vi "detectFly.vi"(4 "focus check":T2=refnum, 5 "im proc controls":T1={"Color Plane"=2, "downsampling"=24, "Filter"=enum."AutoM", "Number of Erosions"=2, "Focus threshold"=20.0, "Focus std threshold"=0.0, "background\nsubtraction"=FALSE, "Threshold"=0} {"Threshold" scale=0.0..255.0; "Color Plane" items=["Red", "Green", "Blue", "Hue", "Saturation", "Luminance", "Value", "Intensity"]}, 6 "processed image container":T2=refnum caption="processed", 7 "cropped image":T2=refnum caption="cropped", 8 "raw image container":T2=refnum caption="raw") -> (0 "acquired FPS":dbl=23.880597014925375, 1 "processed image":T2, 2 "processed FPS":dbl=23.880597014925375, 3 "raw out":T2)   [LabVIEW 2012]
uses:
  <vilib>/vision/Image Controls.llb/IMAQ Image.ctl
  GlobalBaslerCamera.vi
  <vilib>/vision/driver/NI_Vision_Acquisition_Software.lvlib
  <vilib>/vision/NI_Vision_Development_Module.lvlib
panel:
  out "Global Report":T3={"Mean Value"=1.2830653, "Standard Variation"=7.5779014, "Minimal Value"=0.0, "Maximal Value"=151.0, "Area (calibrated)"=1470000.0, "Area (pixels)"=1470000, "%"=100.0, "Calibration Valid"=TRUE} {"Mean Value" format="%.2f"; "%" format="%.2f"; "Area (calibrated)" format="%.2f"; "Maximal Value" format="%.2f"; "Minimal Value" format="%.2f"; "Standard Variation" format="%.2f"}
  out "Buffer Number Out":u32=414
  out "Number of Particles":i32=1
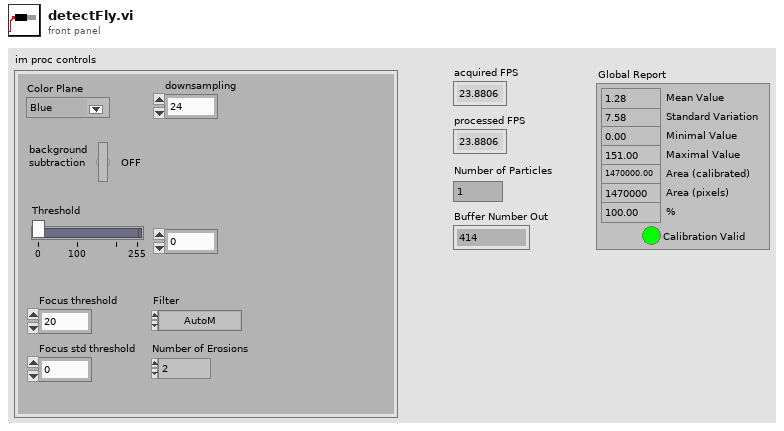
[diagram p1: front panel]
types:
  T1 = cluster{"Color Plane":i32, "downsampling":i32, "Filter":enum32{"AutoM", "Close", "Dilate", "Erode", "Gradient", "Gradient out", "Gradient in", "Hit miss", "Open", "PClose", "POpen", "Thick", "Thin"}, "Number of Erosions":i32, "Focus threshold":sgl, "Focus std threshold":sgl, "background\nsubtraction":bool, "Threshold":u8}
  T2 = typedef "IMAQ Image.ctl" = refnum<image>
  T3 = cluster{"Mean Value":sgl, "Standard Variation":sgl, "Minimal Value":sgl, "Maximal Value":sgl, "Area (calibrated)":sgl, "Area (pixels)":u32, "%":sgl, "Calibration Valid":bool}
  T4 = typedef "IMAQdx.ctl" = refnum<k21>
  T5 = enum32{"Differentiation", "Gradient", "Prewitt", "Roberts", "Sigma", "Sobel"}
  T6 = enum32{"AutoM", "Close", "Dilate", "Erode", "Gradient", "Gradient out", "Gradient in", "Hit miss", "Open", "PClose", "POpen", "Thick", "Thin"}
  T7 = typedef "Particle Parameters" = i32
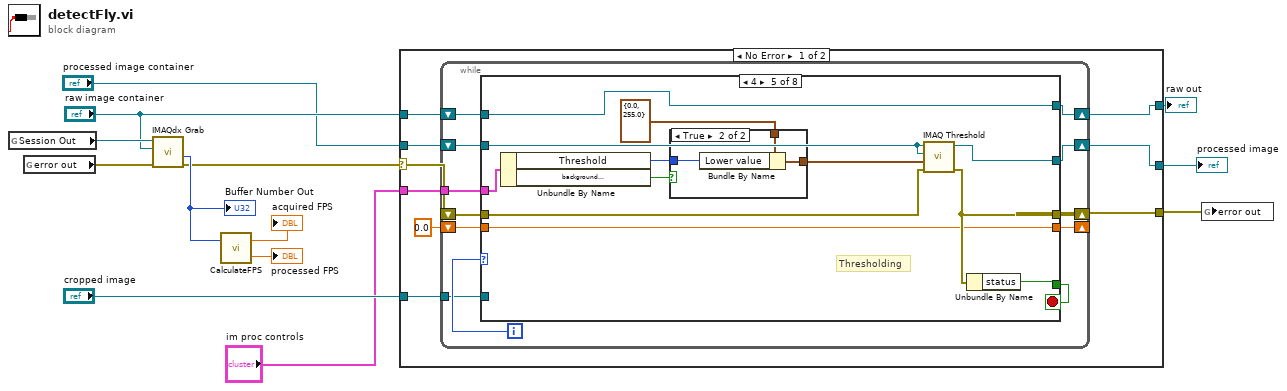
[diagram p0: block diagram]
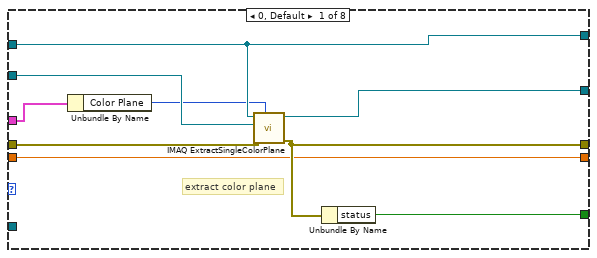
[diagram p2: hidden frame]
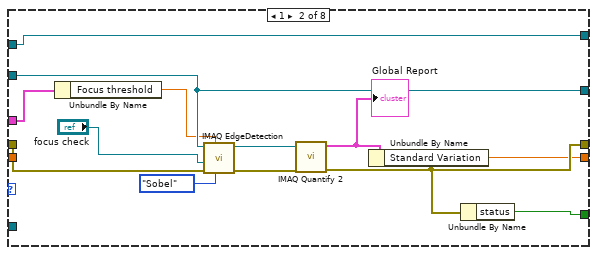
[diagram p3: hidden frame]
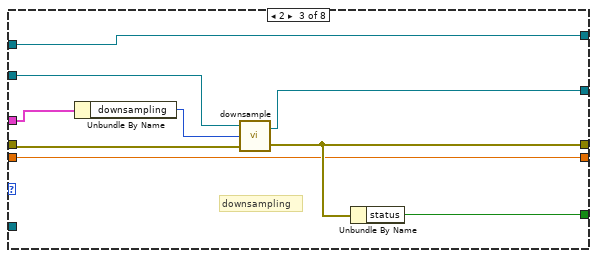
[diagram p4: hidden frame]
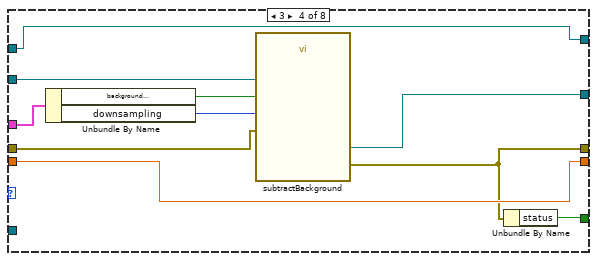
[diagram p5: hidden frame]
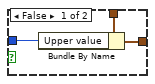
[diagram p6: hidden frame]
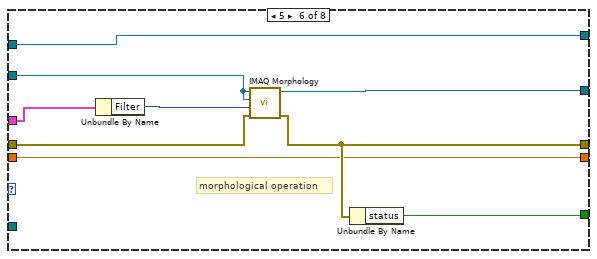
[diagram p7: hidden frame]
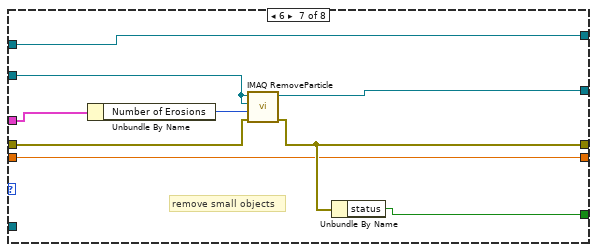
[diagram p8: hidden frame]
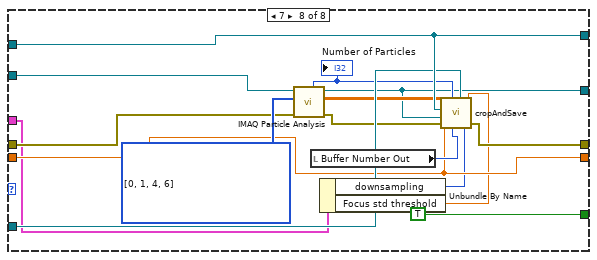
[diagram p9: hidden frame]
diagram:
  n1 = global read "GlobalBaslerCamera.vi" "Session Out"() -> (w13:T4)
  n2 = global read "GlobalBaslerCamera.vi" "error out"() -> (w12:errorcluster)
  n3 = call <vilib>:"IMAQdx Grab.vi"("error in"=w12, "Image In"="raw image container", "Session In"=w13) -> ("error out"=w9:errorcluster, "Buffer Number Out"=w11:u32)  [unwired: 1 in, 6 out]
  "Buffer Number Out" <- w11
  n4 = call "CalculateFPS.vi"("buffer number"=w11) -> ("processed FPS"=→"processed FPS":dbl, "acquired FPS"=→"acquired FPS":dbl)  [unwired: 1 in]
  n5 = case shown="No Error" w9 {
    selector: w9 -> [w22 w129]
    tunnel: "raw image container" -> [w21 w128]
    tunnel: "processed image container" -> [w20 w130]
    tunnel: [w19 w130] -> w6
    tunnel: [w18 w129] -> w4
    tunnel: [w17 w128] -> w5
    tunnel: "cropped image" -> [w16 _]
    tunnel: "im proc controls" -> [w14 _]
    frame No Error {
      n6 = while {
        shift-right: [w32] -> w18
        shift-left: w22 -> [w29]
        tunnel: w16 -> [w27]
        shift-right: [w26] -> _
        shift-left: sgl 0.0 ("Standard Variation") -> [w25]
        tunnel: w14 -> [w24]
        shift-right: [w28] -> w17
        shift-left: w21 -> [w31]
        shift-right: [w23] -> w19
        shift-left: w20 -> [w30]
        i -> [w34]
        stop <- w33 stop-if-true
        n7 = case shown="4" w34 {
          tunnel: [w40 w51 w63 w74 w85 w101 w109 TRUE ("status")] -> w33
          tunnel: [w41 w50 w62 w66 w84 w100 w108 w120] -> w32
          tunnel: w31 -> [w38 w52 w60 w73 w76 w97 w106 w123]
          tunnel: w30 -> [w43 w49 w64 w71 w87 w99 w111 w127]
          tunnel: w29 -> [w42 w47 w65 w68 w86 w102 w110 w125]
          tunnel: [w39 w49 w61 w67 w83 w98 w107 w116] -> w23
          tunnel: [w38 w52 w60 w73 w76 w97 w106 w123] -> w28
          tunnel: w27 -> [_ _ _ _ _ _ _ w122]
          tunnel: [w37 w46 w59 w72 w82 w96 w105 w115] -> w26
          tunnel: w25 -> [w37 _ w59 w72 w82 w96 w105 w115]
          tunnel: w24 -> [w36 w45 w58 w75 w78 w94 w104 w113]
          frame 0, Default {
            # "extract color plane"
            n8 = Unbundle By Name(w36) -> ("Color Plane"=w35:i32)
            n9 = call "IMAQ ExtractSingleColorPlane"("Color Plane"=w35, "error in (no error)"=w42, "Image Dst"=w43, "Image Src"=w38) -> ("error out"=w41:errorcluster, "Image Dst Out"=w39:T2)  [unwired: 6 in]
            n10 = Unbundle By Name(w41) -> ("status"=w40:bool)
          }
          frame 1 {
            n11 = Unbundle By Name(w45) -> ("Focus threshold"=w44:sgl)
            n12 = call "IMAQ EdgeDetection"("Method"=T5."Sobel", "Threshold Value"=w44, "error in (no error)"=w47, "Image Dst"="focus check", "Image Src"=w49) -> ("error out"=w55:errorcluster, "Image Dst Out"=w54:T2)  [unwired: 5 in]
            n13 = call "IMAQ Quantify 2"("error in (no error)"=w55, "Image"=w54) -> ("error out"=w50:errorcluster, "Global Report"=w53:T3)  [unwired: 7 in, 1 out]
            "Global Report" <- w53
            n14 = Unbundle By Name(w53) -> ("Standard Variation"=w46:sgl)
            n15 = Unbundle By Name(w50) -> ("status"=w51:bool)
          }
          frame 2 {
            # "downsampling"
            n16 = Unbundle By Name(w58) -> ("downsampling"=w57:i32)
            n17 = call "downsample.vi"("error in"=w65, "downsampling"=w57, "IMAQImage"=w64) -> ("error out"=w62:errorcluster, "Image Dst Out"=w61:T2)
            n18 = Unbundle By Name(w62) -> ("status"=w63:bool)
          }
          frame 3 {
            n19 = Unbundle By Name(w75) -> ("background\nsubtraction"=w70:bool, "downsampling"=w69:i32)
            n20 = call "subtractBackground.vi"("error IO"=w68, "downsampling"=w69, "saveBG"=w70, "processed image"=w71) -> ("error out"=w66:errorcluster, "processed image out"=w67:T2)  [unwired: 6 in]
            n21 = Unbundle By Name(w66) -> ("status"=w74:bool)
          }
          frame 4 {
            # "Thresholding"
            n22 = Unbundle By Name(w78) -> ("Threshold"=w81:u8, "background\nsubtraction"=w77:bool)
            n23 = case shown="True" w77 {
              tunnel: w81 -> [w90 w93]
              tunnel: [w89 w92] -> w80
              tunnel: cluster{"Lower value":sgl, "Upper value":sgl} {"Lower value"=0.0, "Upper value"=255.0} ("Range") -> [w88 w91]
              frame False {
                n24 = Bundle By Name(cluster=w88, "Upper value"=w90) -> (w89:cluster{"Lower value":sgl, "Upper value":sgl})
              }
              frame True {
                n25 = Bundle By Name(cluster=w91, "Lower value"=w93) -> (w92:cluster{"Lower value":sgl, "Upper value":sgl})
              }
            }
            n26 = call "IMAQ Threshold"("error in (no error)"=w86, "Range"=w80, "Image Dst"=w87, "Image Src"=w87) -> ("error out"=w84:errorcluster, "Image Dst Out"=w83:T2)  [unwired: 6 in]
            n27 = Unbundle By Name(w84) -> ("status"=w85:bool)
          }
          frame 5 {
            # "morphological operation"
            n28 = Unbundle By Name(w94) -> ("Filter"=w95:T6)
            n29 = call "IMAQ Morphology"("error in (no error)"=w102, "Operation"=w95, "Image Dst"=w99, "Image Src"=w99) -> ("error out"=w100:errorcluster, "Image Dst Out"=w98:T2)  [unwired: 6 in]
            n30 = Unbundle By Name(w100) -> ("status"=w101:bool)
          }
          frame 6 {
            # "remove small objects"
            n31 = Unbundle By Name(w104) -> ("Number of Erosions"=w103:i32)
            n32 = call "IMAQ RemoveParticle"("error in (no error)"=w110, "Number of Erosion"=w103, "Image Dst"=w111, "Image Src"=w111) -> ("error out"=w108:errorcluster, "Image Dst Out"=w107:T2)  [unwired: 6 in]
            n33 = Unbundle By Name(w108) -> ("status"=w109:bool)
          }
          frame 7 {
            w126 = T7[] [0, 1, 4, 6] items=["Center of Mass X", "Center of Mass Y", "First Pixel X", "First Pixel Y", "Bounding Rect Left", "Bounding Rect Top", "Bounding Rect Right", "Bounding Rect Bottom", "Max Feret Diameter Start X", "Max Feret Diameter Start Y", "Max Feret Diameter End X", "Max Feret Diameter End Y", "Max Horiz. Segment Length Left", "Max Horiz. Segment Length Right", "Max Horiz. Segment Length Row", "-", "Bounding Rect Width", "Bounding Rect Height", "Bounding Rect Diagonal", "Perimeter", "Convex Hull Perimeter", "Holes' Perimeter", "Max Feret Diameter", "Equivalent Ellipse Major Axis", "Equivalent Ellipse Minor Axis", "Equivalent Ellipse Minor Axis (Feret)", "Equivalent Rect Long Side", "Equivalent Rect Short Side", "Equivalent Rect Diagonal", "Equivalent Rect Short Side (Feret)", "Average Horiz. Segment Length", "Average Vert. Segment Length", "Hydraulic Radius", "Waddel Disk Diameter", "-", "Area", "Holes' Area", "Particle & Holes' Area", "Convex Hull Area", "Image Area", "-", "Number of Holes", "Number of Horiz. Segments", "Number of Vert. Segments", "-", "Orientation", "Max Feret Diameter Orientation", "-", "% Area/Image Area", "% Area/(Particle & Holes' Area)", "Ratio of Equivalent Ellipse Axes", "Ratio of Equivalent Rect Sides", "-", "Elongation Factor", "Compactness Factor", "Heywood Circularity Factor", "Type Factor", "-", "Sum X", "Sum Y", "Sum XX", "Sum XY", "Sum YY", "Sum XXX", "Sum XXY", "Sum XYY", "Sum YYY", "-", "Moment of Inertia XX", "Moment of Inertia XY", "Moment of Inertia YY", "Moment of Inertia XXX", "Moment of Inertia XXY", "Moment of Inertia XYY", "Moment of Inertia YYY", "Norm. Moment of Inertia XX", "Norm. Moment of Inertia XY", "Norm. Moment of Inertia YY", "Norm. Moment of Inertia XXX", "Norm. Moment of Inertia XXY", "Norm. Moment of Inertia XYY", "Norm. Moment of Inertia YYY", "Hu Moment 1", "Hu Moment 2", "Hu Moment 3", "Hu Moment 4", "Hu Moment 5", "Hu Moment 6", "Hu Moment 7"] ("Pixel Measurements")
            n34 = call "IMAQ Particle Analysis"("error in (no error)"=w125, "Pixel Measurements"=w126, "Image"=w127) -> ("error out"=w121:errorcluster, "Particle Measurements (Pixels)"=w119:dbl[][], "Image Out (duplicate)"=w116:T2, "Number of Particles"=w118:i32)  [unwired: 2 in, 3 out]
            "Number of Particles" <- w118
            n35 = local read "Buffer Number Out"() -> (w117:u32)
            n36 = Unbundle By Name(w113) -> ("downsampling"=w114:i32, "Focus std threshold"=w112:sgl)
            n37 = call "cropAndSave.vi"("error in (no error)"=w121, "downsampling"=w114, "std threshold"=w112, "cropped Image"=w122, "buffer number"=w117, "Standard Variation"=w115, "processed image"=w116, "Number of Particles"=w118, "raw image"=w123, "Particle Measurements (Pixels)"=w119) -> ("error out"=w120:errorcluster)
          }
        }
      }
    }
    frame Error {
    }
  }
  "processed image" <- w6
  "raw out" <- w5
  n38 = global write "GlobalBaslerCamera.vi" "error out"(w4) -> ()
